vi "Laser Ablation and Capture.vi"() -> ()   [LabVIEW 2016] (continued)
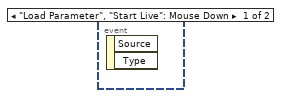
[diagram p2: hidden frame]
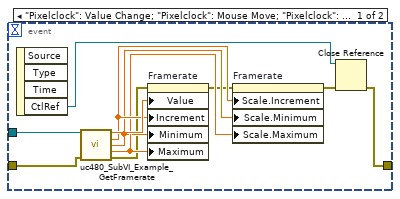
[diagram p3: hidden frame]
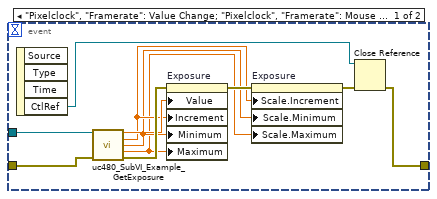
[diagram p4: hidden frame]
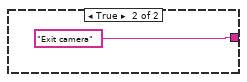
[diagram p5: hidden frame]
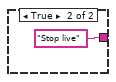
[diagram p6: hidden frame]
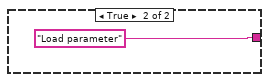
[diagram p7: hidden frame]
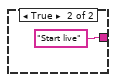
[diagram p8: hidden frame]
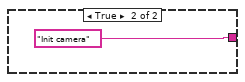
[diagram p9: hidden frame]
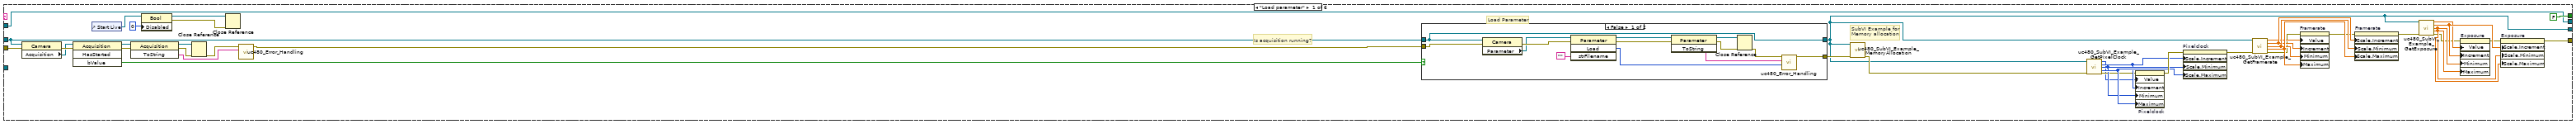
[diagram p10: hidden frame]
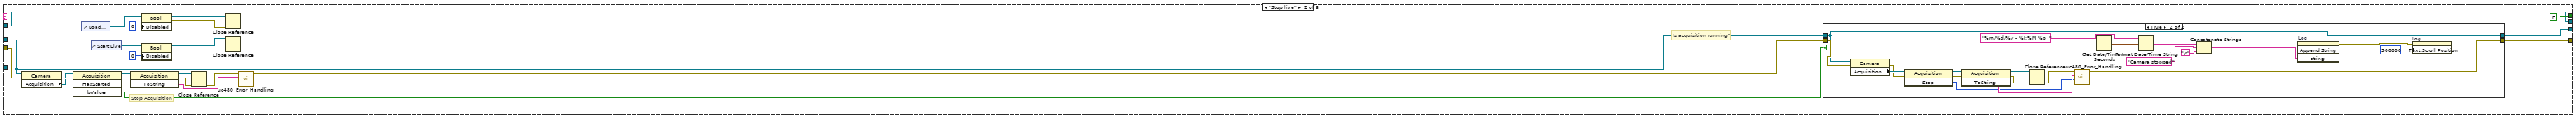
[diagram p12: hidden frame]
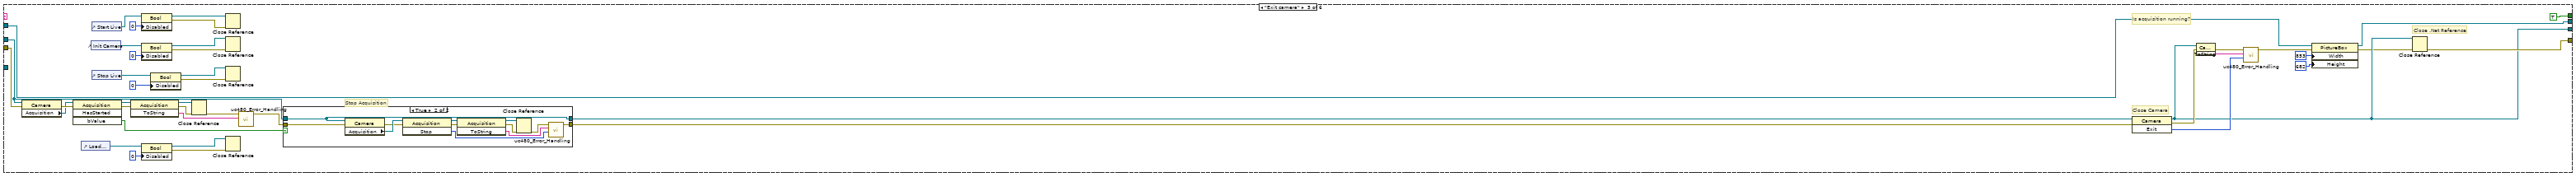
[diagram p14: hidden frame]
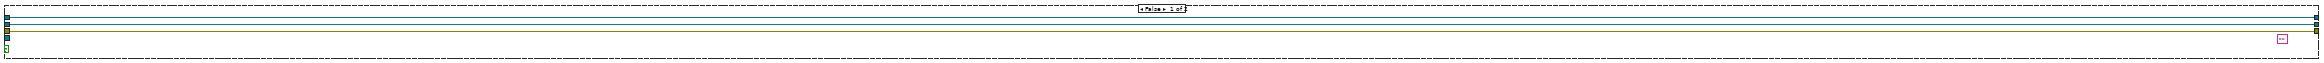
[diagram p16: hidden frame]
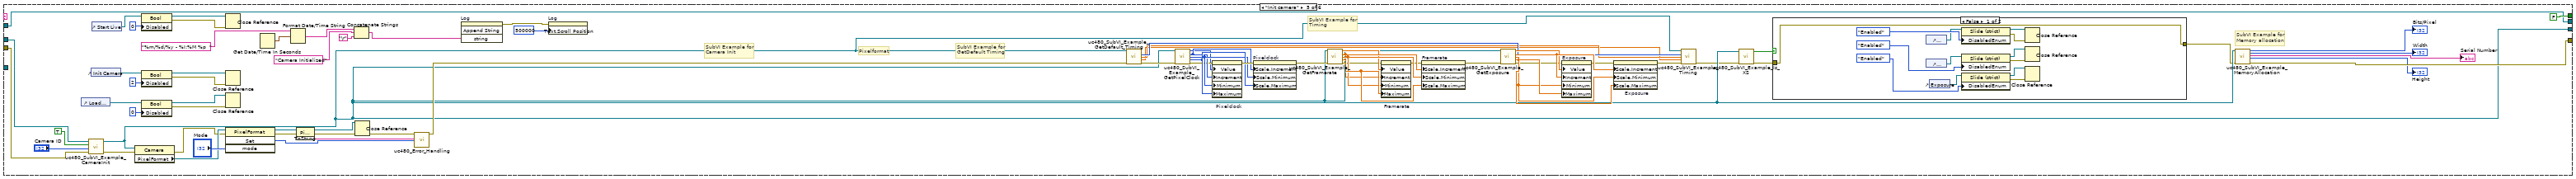
[diagram p18: hidden frame]
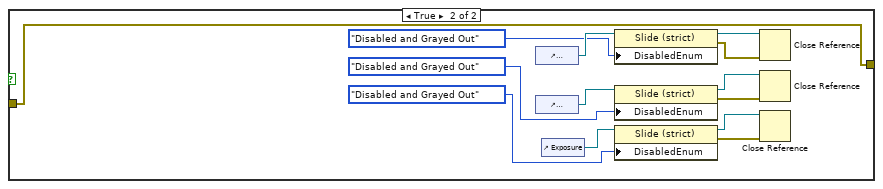
[diagram p19: hidden frame]
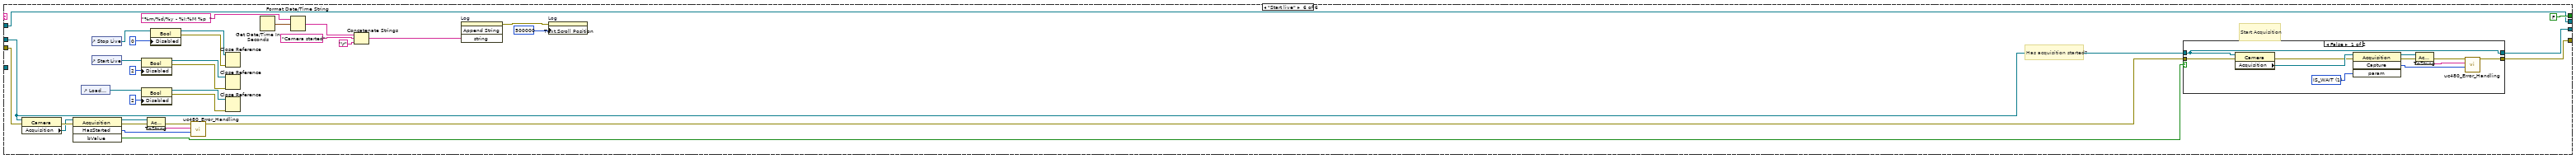
[diagram p20: hidden frame]
            n599 = case shown="False" w1486 {
              tunnel: w1485 -> [w1497 _]
              frame False {
                n600 = call "IMAQ Create"("Image Name"="untitled") -> ("New Image"=w1499:T2)  [unwired: 4 in, 1 out]
                n601 = call "IMAQ ReadFile"("File Path"=w1497, "Image"=w1499) -> ("Image Out"=w1498:T2)  [unwired: 5 in, 4 out]
                n602 = call "IMAQ MaskToROI"("Image"=w1498) -> ("ROI Descriptor"=w1490:T11)  [unwired: 6 in, 2 out]
                n603 = Unbundle By Name(w1490) -> ("Contours"=w1495:T12)  [unwired: 1 out]
                n604 = Index Array(array=w1495) -> (element=w1496:T13)  [unwired: 1 in]
                n605 = Bundle By Name(cluster=w1496, "Type"=u32 6) -> (w1494:T13)
                n606 = Replace Array Subset(array=w1495, new element=w1494) -> (w1493:T12)  [unwired: 1 in]
                n607 = Bundle By Name(cluster=w1490, "Contours"=w1493) -> (w1491:T11)
                n608 = property on="Source" class="ImageControl"("ROI"=w1491) -> ()  [unwired: 2 in, 2 out]
              }
              frame True {
              }
            }
          }
        }
      }
      event "Axes Manual Control": Value Change {
        n609 = event-data() -> ()  [unwired: 1 in, 6 out]
        n610 = case shown="True" "Axes Manual Control" {
          tunnel: w1503 -> [_ w1515]
          tunnel: w1502 -> [_ w1514]
          tunnel: w1501 -> [_ w1513]
          frame False {
          }
          frame True {
            n611 = flat-sequence {
              tunnel: w1515 -> [w1525]
              tunnel: w1514 -> [w1524]
              tunnel: w1513 -> [w1523]
              tunnel: [w1525] -> w1512
              tunnel: [w1524] -> w1511
              tunnel: [w1523] -> w1510
              tunnel: [w1522] -> w1509
              tunnel: [w1521] -> w1508
              tunnel: [w1520] -> w1507
              tunnel: [w1519] -> w1506
              tunnel: w1512 -> [w1568]
              tunnel: w1511 -> [w1567]
              tunnel: w1510 -> [w1566]
              tunnel: w1509 -> [w1561]
              tunnel: w1508 -> [w1560]
              tunnel: w1507 -> [w1551]
              tunnel: w1506 -> [w1550]
              frame #0 {
                n612 = call <userlib>:"Open TCP-IP.vi"("IP address"=w1525) -> ("error out"=w1517:errorcluster, "Connection ID"=w1526:T9)  [unwired: 8 in, 1 out]
                n613 = call <vilib>:"Simple Error Handler.vi"("error in (no error)"=w1517) -> ("error?"=w1516:bool, "error out"=w1518:errorcluster)  [unwired: 4 in, 3 out]
                n614 = case shown="True" w1516 {
                  tunnel: w1526 -> [w1541 _]
                  tunnel: w1518 -> [w1540 _]
                  tunnel: w1524 -> [w1537 _]
                  tunnel: w1523 -> [w1536 _]
                  tunnel: [w1535 w1545] -> w1522
                  tunnel: [w1534 w1545] -> w1521
                  tunnel: [w1530 w1544] -> w1520
                  tunnel: [w1529 w1544] -> w1519
                  frame False {
                    n615 = call "Get Stages Status.vi"("error in (no error)"=w1540, "Group Name (250 c max)"=w1537, "connection ID in"=w1541) -> ("error out"=w1539:errorcluster, "XPS error out"=w1538:errorcluster, "Group Status String"=w1534:string, "connection ID out"=w1533:T9, "Status"=w1529:i32)  [unwired: 4 in]
                    n616 = call "Get Stages Status.vi"("error in (no error)"=w1539, "XPS error in (no error)"=w1538, "Group Name (250 c max)"=w1536, "connection ID in"=w1533) -> ("error out"=w1543:errorcluster, "XPS error out"=w1532:errorcluster, "Group Status String"=w1535:string, "connection ID out"=w1542:T9, "Status"=w1530:i32)  [unwired: 3 in]
                    n617 = call <vilib>:"Simple Error Handler.vi"("error source (\" \")"="Axis manual control check" ("error source (\" \")"), "error in (no error)"=w1532) -> ()  [unwired: 3 in, 5 out]
                    n618 = call <userlib>:"Close TCP-IP.vi"("error in (no error)"=w1543, "connection ID in"=w1542) -> ("Error out"=w1531:errorcluster)  [unwired: 9 in]
                    n619 = call <vilib>:"Simple Error Handler.vi"("error source (\" \")"="TCP close Axis manual control check" ("error source (\" \")"), "error in (no error)"=w1531) -> ()  [unwired: 3 in, 5 out]
                  }
                  frame True {
                    w1544 = 0
                    w1545 = ""
                  }
                }
              }
              frame #1 {
                w1554 = 47 ("y")
                w1555 = "Ready"
                n620 = String Subset(string=w1560, offset (0)=0, length (rest)=5 ("length (rest)")) -> (substring=w1557:string)
                n621 = String Subset(string=w1561, offset (0)=0, length (rest)=5 ("length (rest)")) -> (substring=w1556:string)
                n622 = Equal?(x=w1557, y=w1555) -> (x = y?=w1558:bool)
                n623 = Equal?(x=w1555, y=w1556) -> (x = y?=w1559:bool)
                n624 = Equal?(x=w1554, y=w1550) -> (x = y?=w1552:bool)
                n625 = Equal?(x=w1551, y=w1554) -> (x = y?=w1553:bool)
                n626 = And(x=w1553, y=w1552) -> (x .and. y?=w1547:bool)
                n627 = And(x=w1558, y=w1559) -> (x .and. y?=w1548:bool)
                n628 = Not(x=w1547) -> (.not. x?=w1546:bool)
                n629 = And(x=w1548, y=w1546) -> (x .and. y?=w1549:bool)
                n630 = case shown="True" w1549 {
                  tunnel: w1568 -> [_ w1576]
                  tunnel: w1567 -> [_ w1575]
                  tunnel: w1566 -> [_ w1574]
                  tunnel: w1546 -> [w1569 _]
                  frame False {
                    n631 = case shown="False" w1569 {
                      frame False {
                        n632 = One Button Dialog(message="One or more axis already in jogging position") -> ()  [unwired: 1 in, 1 out]
                      }
                      frame True {
                        n633 = One Button Dialog(message="Axes are not ready") -> ()  [unwired: 1 in, 1 out]
                      }
                    }
                  }
                  frame True {
                    n634 = local read "Axis 2 inverted?"() -> (w1573:bool)
                    n635 = local read "Axis 1 inverted?"() -> (w1572:bool)
                    n636 = call "XPS Controller.vi"("Axis 2"=w1574, "Axis 1"=w1575, "Controller Address"=w1576, "Axis 2 \ninverted?"=w1573, "Axis 1 \ninverted?"=w1572) -> ()  [unwired: 6 in]
                  }
                }
              }
            }
          }
        }
      }
      event "Home Axes": Value Change {
        n637 = event-data() -> ()  [unwired: 1 in, 6 out]
        n638 = flat-sequence {
          tunnel: w1583 -> [w1589]
          tunnel: w1584 -> [w1590]
          tunnel: w1585 -> [w1591]
          tunnel: "Home Axes" -> [w1592]
          tunnel: [w1592] -> w1581
          tunnel: [w1591] -> w1580
          tunnel: [w1590] -> w1579
          tunnel: [w1589] -> w1578
          tunnel: [w1588] -> w1577
          tunnel: [w1596] -> w1582
          tunnel: w1581 -> [w1594]
          tunnel: w1580 -> [w1599]
          tunnel: w1579 -> [w1597]
          tunnel: w1578 -> [w1598]
          tunnel: w1577 -> [w1595]
          tunnel: [w1678] -> w1586
          tunnel: w1582 -> [w1677]
          frame #0 {
            n639 = call "Display Message to User"() -> ("OK"=w1588:bool)  [unwired: 10 in, 1 out]
          }
          frame #1 {
            n640 = And(x=w1594, y=w1595) -> (x .and. y?=w1593:bool)
            n641 = case shown="True" w1593 {
              tunnel: w1599 -> [_ w1615]
              tunnel: w1597 -> [_ w1616]
              tunnel: w1598 -> [_ w1613]
              tunnel: w1597 -> [_ w1614]
              tunnel: [FALSE w1606] -> w1596
              frame False {
              }
              frame True {
                w1612 = 47 ("y")
                w1628 = "Ready"
                n642 = call <userlib>:"Open TCP-IP.vi"("IP address"=w1615) -> ("error out"=w1601:errorcluster, "Connection ID"=w1619:T9)  [unwired: 8 in, 1 out]
                n643 = call <vilib>:"Simple Error Handler.vi"("error in (no error)"=w1601) -> ("error?"=w1603:bool, "error out"=w1602:errorcluster)  [unwired: 4 in, 3 out]
                n644 = case shown="False" w1603 {
                  tunnel: w1602 -> [w1642 _]
                  tunnel: w1619 -> [w1641 _]
                  tunnel: [w1638 w1647] -> w1618
                  tunnel: [w1637 w1647] -> w1617
                  tunnel: w1616 -> [w1636 _]
                  tunnel: w1613 -> [w1635 _]
                  tunnel: [w1632 w1646] -> w1611
                  tunnel: [w1631 w1646] -> w1610
                  frame False {
                    n645 = call "Get Stages Status.vi"("error in (no error)"=w1642, "Group Name (250 c max)"=w1636, "connection ID in"=w1641) -> ("error out"=w1643:errorcluster, "XPS error out"=w1644:errorcluster, "Group Status String"=w1638:string, "connection ID out"=w1645:T9, "Status"=w1631:i32)  [unwired: 4 in]
                    n646 = call "Get Stages Status.vi"("error in (no error)"=w1643, "XPS error in (no error)"=w1644, "Group Name (250 c max)"=w1635, "connection ID in"=w1645) -> ("error out"=w1639:errorcluster, "XPS error out"=w1634:errorcluster, "Group Status String"=w1637:string, "connection ID out"=w1640:T9, "Status"=w1632:i32)  [unwired: 3 in]
                    n647 = call <vilib>:"Simple Error Handler.vi"("error source (\" \")"="home axis check" ("error source (\" \")"), "error in (no error)"=w1634) -> ()  [unwired: 3 in, 5 out]
                    n648 = call <userlib>:"Close TCP-IP.vi"("error in (no error)"=w1639, "connection ID in"=w1640) -> ("Error out"=w1633:errorcluster)  [unwired: 9 in]
                    n649 = call <vilib>:"Simple Error Handler.vi"("error source (\" \")"="TCP close home axis check" ("error source (\" \")"), "error in (no error)"=w1633) -> ()  [unwired: 3 in, 5 out]
                  }
                  frame True {
                    w1646 = 0
                    w1647 = ""
                  }
                }
                n650 = Equal?(x=w1612, y=w1610) -> (x = y?=w1609:bool)
                n651 = Equal?(x=w1611, y=w1612) -> (x = y?=w1608:bool)
                n652 = String Subset(string=w1618, offset (0)=0, length (rest)=5 ("length (rest)")) -> (substring=w1626:string)
                n653 = String Subset(string=w1617, offset (0)=0, length (rest)=5 ("length (rest)")) -> (substring=w1627:string)
                n654 = Equal?(x=w1626, y=w1628) -> (x = y?=w1625:bool)
                n655 = Equal?(x=w1628, y=w1627) -> (x = y?=w1624:bool)
                n656 = And(x=w1608, y=w1609) -> (x .and. y?=w1604:bool)
                n657 = Not(x=w1604) -> (.not. x?=w1605:bool)
                n658 = And(x=w1625, y=w1624) -> (x .and. y?=w1607:bool)
                n659 = And(x=w1607, y=w1605) -> (x .and. y?=w1606:bool)
                n660 = case shown="True" w1606 {
                  tunnel: w1615 -> [_ w1657]
                  tunnel: w1614 -> [_ w1656]
                  tunnel: w1613 -> [_ w1655]
                  tunnel: w1604 -> [w1648 _]
                  frame False {
                    n661 = case shown="True" w1648 {
                      frame False {
                        n662 = One Button Dialog(message="Axes are not ready") -> ()  [unwired: 1 in, 1 out]
                      }
                      frame True {
                        n663 = One Button Dialog(message="One or more axis are in jogging mode") -> ()  [unwired: 1 in, 1 out]
                      }
                    }
                  }
                  frame True {
                    n664 = call <userlib>:"Open TCP-IP.vi"("IP address"=w1657) -> ("error out"=w1673:errorcluster, "Connection ID"=w1674:T9)  [unwired: 8 in, 1 out]
                    n665 = call <userlib>:"Group Kill.vi"("error in (no error)"=w1673, "Group Name (250 c max)"=w1656, "connection ID in"=w1674) -> ("error out"=w1671:errorcluster, "XPS error out"=w1672:errorcluster, "connection ID out"=w1668:T9)  [unwired: 6 in]
                    n666 = call <userlib>:"Group Initialize.vi"("error in (no error)"=w1671, "XPS error in (no error)"=w1672, "Group Name (250 c max)"=w1656, "connection ID in"=w1668) -> ("error out"=w1669:errorcluster, "XPS error out"=w1670:errorcluster, "connection ID out"=w1667:T9)  [unwired: 5 in]
                    n667 = call <userlib>:"Group Home Search.vi"("error in (no error)"=w1669, "XPS error in (no error)"=w1670, "Group Name (250 c max)"=w1656, "connection ID in"=w1667) -> ("error out"=w1658:errorcluster, "XPS error out"=w1659:errorcluster, "connection ID out"=w1666:T9)  [unwired: 5 in]
                    n668 = call <userlib>:"Group Kill.vi"("error in (no error)"=w1658, "XPS error in (no error)"=w1659, "Group Name (250 c max)"=w1655, "connection ID in"=w1666) -> ("error out"=w1660:errorcluster, "XPS error out"=w1661:errorcluster, "connection ID out"=w1665:T9)  [unwired: 5 in]
                    n669 = call <userlib>:"Group Initialize.vi"("error in (no error)"=w1660, "XPS error in (no error)"=w1661, "Group Name (250 c max)"=w1655, "connection ID in"=w1665) -> ("error out"=w1662:errorcluster, "XPS error out"=w1663:errorcluster, "connection ID out"=w1664:T9)  [unwired: 5 in]
                    n670 = call <userlib>:"Group Home Search.vi"("error in (no error)"=w1662, "XPS error in (no error)"=w1663, "Group Name (250 c max)"=w1655, "connection ID in"=w1664) -> ("error out"=w1675:errorcluster, "XPS error out"=w1654:errorcluster, "connection ID out"=w1676:T9)  [unwired: 5 in]
                    n671 = call <vilib>:"Simple Error Handler.vi"("error source (\" \")"="home axis " ("error source (\" \")"), "error in (no error)"=w1654) -> ()  [unwired: 3 in, 5 out]
                    n672 = call <userlib>:"Close TCP-IP.vi"("error in (no error)"=w1675, "connection ID in"=w1676) -> ("Error out"=w1653:errorcluster)  [unwired: 9 in]
                    n673 = call <vilib>:"Simple Error Handler.vi"("error source (\" \")"="TCP close home axis " ("error source (\" \")"), "error in (no error)"=w1653) -> ()  [unwired: 3 in, 5 out]
                  }
                }
              }
            }
          }
          frame #2 {
            n674 = case shown="True" w1677 {
              tunnel: ["" ("StringOut") "Axes have been moved to home position" ("StringOut")] -> w1678
              frame False {
              }
              frame True {
              }
            }
          }
        }
      }
      event "Transparency": Value Change {
        n675 = event-data() -> ()  [unwired: 1 in, 6 out]
        n676 = control-ref of="This VI"() -> (w1682:refnum<vi>)
        n677 = property class="VI"(reference=w1682, "FP:Transparency"="Transparency") -> ()  [unwired: 1 in, 2 out]
      }
      event "Capture": Value Change {
        w1683 = 47 ("y")
        w1709 = "Ready"
        n678 = event-data() -> ()  [unwired: 1 in, 6 out]
        n679 = call <userlib>:"Open TCP-IP.vi"("IP address"=w1697) -> ("error out"=w1686:errorcluster, "Connection ID"=w1700:T9)  [unwired: 8 in, 1 out]
        n680 = call <vilib>:"Simple Error Handler.vi"("error in (no error)"=w1686) -> ("error?"=w1684:bool, "error out"=w1685:errorcluster)  [unwired: 4 in, 3 out]
        n681 = case shown="False" w1684 {
          tunnel: w1685 -> [w1723 _]
          tunnel: w1700 -> [w1722 _]
          tunnel: [w1719 w1727] -> w1699
          tunnel: [w1718 w1727] -> w1698
          tunnel: w1696 -> [w1717 _]
          tunnel: w1695 -> [w1716 _]
          tunnel: [w1714 w1728] -> w1694
          tunnel: [w1713 w1728] -> w1693
          frame False {
            n682 = call "Get Stages Status.vi"("error in (no error)"=w1723, "Group Name (250 c max)"=w1717, "connection ID in"=w1722) -> ("error out"=w1724:errorcluster, "XPS error out"=w1725:errorcluster, "Group Status String"=w1719:string, "connection ID out"=w1726:T9, "Status"=w1713:i32)  [unwired: 4 in]
            n683 = call "Get Stages Status.vi"("error in (no error)"=w1724, "XPS error in (no error)"=w1725, "Group Name (250 c max)"=w1716, "connection ID in"=w1726) -> ("error out"=w1720:errorcluster, "XPS error out"=w1715:errorcluster, "Group Status String"=w1718:string, "connection ID out"=w1721:T9, "Status"=w1714:i32)  [unwired: 3 in]
            n684 = call <vilib>:"Simple Error Handler.vi"("error source (\" \")"="Capture check" ("error source (\" \")"), "error in (no error)"=w1715) -> ()  [unwired: 3 in, 5 out]
            n685 = call <userlib>:"Close TCP-IP.vi"("error in (no error)"=w1720, "connection ID in"=w1721) -> ("Error out"=w1711:errorcluster)  [unwired: 9 in]
            n686 = call <vilib>:"Simple Error Handler.vi"("error in (no error)"=w1711) -> ()  [unwired: 4 in, 5 out]
          }
          frame True {
            w1728 = 0
            w1727 = ""
          }
        }
        n687 = Equal?(x=w1694, y=w1683) -> (x = y?=w1692:bool)
        n688 = Equal?(x=w1683, y=w1693) -> (x = y?=w1691:bool)
        n689 = String Subset(string=w1699, offset (0)=0, length (rest)=5 ("length (rest)")) -> (substring=w1707:string)
        n690 = String Subset(string=w1698, offset (0)=0, length (rest)=5 ("length (rest)")) -> (substring=w1708:string)
        n691 = Equal?(x=w1707, y=w1709) -> (x = y?=w1706:bool)
        n692 = Equal?(x=w1709, y=w1708) -> (x = y?=w1705:bool)
        n693 = And(x=w1692, y=w1691) -> (x .and. y?=w1688:bool)
        n694 = Not(x=w1688) -> (.not. x?=w1687:bool)
        n695 = And(x=w1706, y=w1705) -> (x .and. y?=w1690:bool)
        n696 = And(x=w1690, y=w1687) -> (x .and. y?=w1689:bool)
        n697 = case shown="True" w1689 {
          tunnel: ["" w1754] -> w1710
          tunnel: w1697 -> [_ w1753]
          tunnel: w1695 -> [_ w1752]
          tunnel: w1696 -> [_ w1751]
          tunnel: w1688 -> [w1729 _]
          frame False {
            n698 = case shown="True" w1729 {
              frame False {
                n699 = One Button Dialog(message="Axes are not ready") -> ()  [unwired: 1 in, 1 out]
              }
              frame True {
                n700 = One Button Dialog(message="One or more axis are in jogging mode") -> ()  [unwired: 1 in, 1 out]
              }
            }
          }
          frame True {
            n701 = flat-sequence {
              tunnel: [w1784] -> w1765
              tunnel: [w1770] -> w1764
              tunnel: [w1769] -> w1763
              tunnel: [w1783] -> w1762
              tunnel: [w1782] -> w1761
              tunnel: [w1781] -> w1760
              tunnel: [w1768] -> w1759
              tunnel: w1751 -> [w1779]
              tunnel: w1752 -> [w1780]
              tunnel: w1753 -> [w1768]
              tunnel: [w1767] -> w1740
              tunnel: [w1766] -> w1736
              tunnel: w1765 -> [w1804]
              tunnel: w1764 -> [w1792]
              tunnel: w1763 -> [w1791]
              tunnel: w1762 -> [w1802]
              tunnel: w1761 -> [w1801]
              tunnel: [w1796] -> w1758
              tunnel: w1760 -> [w1796]
              tunnel: [w1795] -> w1757
              tunnel: w1759 -> [w1795]
              tunnel: [w1792] -> w1750
              tunnel: [w1791] -> w1748
              tunnel: [w1790] -> w1741
              tunnel: w1740 -> [w1790]
              tunnel: [w1789] -> w1737
              tunnel: w1736 -> [w1789]
              tunnel: [w1810] -> w1756
              tunnel: w1758 -> [w1810]
              tunnel: [w1809] -> w1755
              tunnel: w1757 -> [w1809]
              tunnel: w1750 -> [w1808]
              tunnel: [w1808] -> w1749
              tunnel: w1748 -> [w1807]
              tunnel: [w1807] -> w1747
              tunnel: [w1806] -> w1742
              tunnel: w1741 -> [w1806]
              tunnel: [w1805] -> w1738
              tunnel: w1737 -> [w1805]
              tunnel: w1756 -> [w1824]
              tunnel: w1755 -> [w1814]
              tunnel: [w1823] -> w1746
              tunnel: w1749 -> [w1813]
              tunnel: w1747 -> [w1812]
              tunnel: [w1817] -> w1744
              tunnel: [w1816] -> w1743
              tunnel: w1742 -> [w1816]
              tunnel: [w1815] -> w1739
              tunnel: w1738 -> [w1815]
              tunnel: [w1814] -> w1735
              tunnel: [w1813] -> w1734
              tunnel: [w1812] -> w1733
              tunnel: w1746 -> [w1846]
              tunnel: [w1846] -> w1745
              tunnel: w1744 -> [w1842]
              tunnel: w1743 -> [w1836]
              tunnel: w1739 -> [w1835]
              tunnel: w1735 -> [w1840]
              tunnel: w1734 -> [w1834]
              tunnel: w1733 -> [w1833]
              tunnel: [w1851] -> w1754
              tunnel: w1745 -> [w1848]
              frame #0 {
                w1788 = ".Pos"
                n702 = call <userlib>:"Open TCP-IP.vi"("IP address"=w1768) -> ("error out"=w1773:errorcluster, "Connection ID"=w1775:T9)  [unwired: 5 in, 4 out]
                n703 = Concatenate Strings(w1780, w1788) -> (w1769:string)
                n704 = Concatenate Strings(w1779, w1788) -> (w1770:string)
                n705 = call <userlib>:"Single Axis Group Position Current Get.vi"("error in (no error)"=w1773, "SingleAxis Group  Name (250 c max)"=w1770, "connection ID in"=w1775) -> ("error out"=w1776:errorcluster, "XPS error out"=w1777:errorcluster, "Current Position (units)"=w1766:dbl, "connection ID out"=w1778:T9)  [unwired: 5 in]
                "Pre-Capture Axis 1" <- w1766
                n706 = call <userlib>:"Single Axis Group Position Current Get.vi"("error in (no error)"=w1776, "XPS error in (no error)"=w1777, "SingleAxis Group  Name (250 c max)"=w1769, "connection ID in"=w1778) -> ("error out"=w1772:errorcluster, "XPS error out"=w1771:errorcluster, "Current Position (units)"=w1767:dbl, "connection ID out"=w1774:T9)  [unwired: 4 in]
                "Pre-Capture Axis 2" <- w1767
                n707 = local read "Axis Initial Parameters"() -> (w1781:T1)
                n708 = call <userlib>:"Positioner SGamma Parameters Set.vi"("SGamma Parameters"=w1781, "error in (no error)"=w1772, "XPS error in (no error)"=w1771, "Positioner Name (250 c max)"=w1770, "connection ID in"=w1774) -> ("error out"=w1785:errorcluster, "XPS error out"=w1786:errorcluster, "connection ID out"=w1787:T9)  [unwired: 4 in]
                n709 = call <userlib>:"Positioner SGamma Parameters Set.vi"("SGamma Parameters"=w1781, "error in (no error)"=w1785, "XPS error in (no error)"=w1786, "Positioner Name (250 c max)"=w1769, "connection ID in"=w1787) -> ("error out"=w1783:errorcluster, "XPS error out"=w1782:errorcluster, "connection ID out"=w1784:T9)  [unwired: 4 in]
              }
              frame #1 {
                n710 = local read "Axis 1 Offset"() -> (w1794:dbl)
                n711 = local read "Axis 2 Offset"() -> (w1793:dbl)
                n712 = call <userlib>:"Single Axis Group Move Relative.vi"("Target Displacement (units)"=w1794, "error in (no error)"=w1802, "XPS error in (no error)"=w1801, "SingleAxis Group  Name (250 c max)"=w1792, "connection ID in"=w1804) -> ("error out"=w1799:errorcluster, "XPS error out"=w1800:errorcluster, "connection ID out"=w1803:T9)  [unwired: 4 in]
                n713 = call <userlib>:"Single Axis Group Move Relative.vi"("Target Displacement (units)"=w1793, "error in (no error)"=w1799, "XPS error in (no error)"=w1800, "SingleAxis Group  Name (250 c max)"=w1791, "connection ID in"=w1803) -> ("error out"=w1797:errorcluster, "connection ID out"=w1798:T9)  [unwired: 4 in, 1 out]
                n714 = call <userlib>:"Close TCP-IP.vi"("error in (no error)"=w1797, "connection ID in"=w1798) -> ()  [unwired: 9 in, 1 out]
              }
              frame #2 {
                n715 = Wait (ms)(milliseconds to wait=u32 1000) -> ()  [unwired: 1 out]
              }
              frame #3 {
                n716 = local read "Speed (µm/s)"() -> (w1828:i32)
                n717 = local read "Processi time (sec)"() -> (w1822:i32)
                n718 = local read "Laser on/off array"() -> (w1831:bool[][])
                n719 = local read "Commands array"() -> (w1832:string[][])
                n720 = local read "ROI Area \n(mm2)"() -> (w1820:dbl)
                n721 = local read "Laser Com Delay"() -> (w1819:i32)
                n722 = local read "VISA Laser port"() -> (w1818:string)
                n723 = Divide(x=w1828, y=1000) -> (x/y=w1825:dbl)
                n724 = call "Capture.vi"("Commands array"=w1832, "XPS_Address"=w1814, "VISA resource name"=w1818, "laser array index"=0, "Process time"=w1822, "Axis Speed"=w1825, "Laser on/off array"=w1831, "stop"=FALSE ("STOP CAPTURE"), "delay before read (ms)"=w1819, "Axis Initial Parameters"=w1824, "ROI Area \n(mm2)"=w1820, "Axis 2"=w1812, "Axis 1"=w1813, "OPO on?"=TRUE, "Acceleration (units/seconds²)"="Acceleration \n(mm/s²)") -> ("Elapsed time"=w1823:dbl, "XPS error out"=w1817:errorcluster)  [unwired: 2 in, 1 out]
              }
              frame #4 {
                n725 = call <userlib>:"Open TCP-IP.vi"("IP address"=w1840) -> ("error out"=w1839:errorcluster, "Connection ID"=w1841:T9)  [unwired: 5 in, 4 out]
                n726 = call <userlib>:"Single Axis Group Move Absolute.vi"("Target Position (units)"=w1835, "error in (no error)"=w1839, "XPS error in (no error)"=w1842, "SingleAxis Group  Name (250 c max)"=w1834, "connection ID in"=w1841) -> ("error out"=w1844:errorcluster, "XPS error out"=w1843:errorcluster, "connection ID out"=w1845:T9)  [unwired: 4 in]
                n727 = call <userlib>:"Single Axis Group Move Absolute.vi"("Target Position (units)"=w1836, "error in (no error)"=w1844, "XPS error in (no error)"=w1843, "SingleAxis Group  Name (250 c max)"=w1833, "connection ID in"=w1845) -> ("error out"=w1837:errorcluster, "connection ID out"=w1838:T9)  [unwired: 4 in, 1 out]
                n728 = call <userlib>:"Close TCP-IP.vi"("error in (no error)"=w1837, "connection ID in"=w1838) -> ()  [unwired: 9 in, 1 out]
              }
              frame #5 {
                n729 = Number To Decimal String(number=w1848) -> (decimal integer string=w1847:string)  [unwired: 1 in]
                n730 = Concatenate Strings("Capture completed in " ("StringOut"), w1847, " seconds" ("string")) -> (w1851:string)
              }
            }
          }
        }
      }
      event "Microscope/Capture \nstatus button": Value Change {
        w1871 = 47 ("y")
        w1884 = "Ready"
        n731 = event-data() -> ()  [unwired: 1 in, 6 out]
        n732 = call <userlib>:"Open TCP-IP.vi"("IP address"=w1854) -> ("error out"=w1887:errorcluster, "Connection ID"=w1888:T9)  [unwired: 8 in, 1 out]
        n733 = call <vilib>:"Simple Error Handler.vi"("error in (no error)"=w1887) -> ("error?"=w1885:bool, "error out"=w1886:errorcluster)  [unwired: 4 in, 3 out]
        n734 = case shown="False" w1885 {
          tunnel: w1888 -> [w1966 _]
          tunnel: [w1963 w1970] -> w1870
          tunnel: [w1962 w1970] -> w1869
          tunnel: w1864 -> [w1961 _]
          tunnel: w1865 -> [w1960 _]
          tunnel: [w1958 w1971] -> w1868
          tunnel: [w1957 w1971] -> w1867
          tunnel: w1886 -> [w1954 _]
          frame False {
            n735 = call "Get Stages Status.vi"("error in (no error)"=w1954, "Group Name (250 c max)"=w1961, "connection ID in"=w1966) -> ("error out"=w1967:errorcluster, "XPS error out"=w1968:errorcluster, "Group Status String"=w1963:string, "connection ID out"=w1969:T9, "Status"=w1957:i32)  [unwired: 4 in]
            n736 = call "Get Stages Status.vi"("error in (no error)"=w1967, "XPS error in (no error)"=w1968, "Group Name (250 c max)"=w1960, "connection ID in"=w1969) -> ("error out"=w1964:errorcluster, "XPS error out"=w1959:errorcluster, "Group Status String"=w1962:string, "connection ID out"=w1965:T9, "Status"=w1958:i32)  [unwired: 3 in]
            n737 = call <vilib>:"Simple Error Handler.vi"("error source (\" \")"="Axes check" ("error source (\" \")"), "error in (no error)"=w1959) -> ()  [unwired: 3 in, 5 out]
            n738 = call <userlib>:"Close TCP-IP.vi"("error in (no error)"=w1964, "connection ID in"=w1965) -> ("Error out"=w1955:errorcluster)  [unwired: 9 in]
            n739 = call <vilib>:"Simple Error Handler.vi"("error in (no error)"=w1955) -> ()  [unwired: 4 in, 5 out]
          }
          frame True {
            w1971 = 0
            w1970 = ""
          }
        }
        n740 = Equal?(x=w1868, y=w1871) -> (x = y?=w1875:bool)
        n741 = Equal?(x=w1871, y=w1867) -> (x = y?=w1874:bool)
        n742 = String Subset(string=w1870, offset (0)=0, length (rest)=5 ("length (rest)")) -> (substring=w1882:string)
        n743 = String Subset(string=w1869, offset (0)=0, length (rest)=5 ("length (rest)")) -> (substring=w1883:string)
        n744 = case shown="False" "Microscope/Capture \nstatus button" {
          tunnel: ["capture " "microscope "] -> w1858
          frame False {
          }
          frame True {
          }
        }
        n745 = Equal?(x=w1882, y=w1884) -> (x = y?=w1881:bool)
        n746 = Equal?(x=w1884, y=w1883) -> (x = y?=w1880:bool)
        n747 = And(x=w1875, y=w1874) -> (x .and. y?=w1866:bool)
        n748 = Not(x=w1866) -> (.not. x?=w1872:bool)
        n749 = And(x=w1881, y=w1880) -> (x .and. y?=w1873:bool)
        n750 = And(x=w1873, y=w1872) -> (x .and. y?=w1856:bool)
        n751 = Concatenate Strings("Do you want to move the axis to the " ("message"), w1858, "position?" ("string")) -> (w1857:string)
        n752 = Two Button Dialog(message=w1857, 1:"No" ("F button name (\"Cancel\")"), 2:"Yes" ("T button name (\"OK\")")) -> (T button?=w1853:bool)
        n753 = case shown="False" w1853 {
          tunnel: "Microscope/Capture \nstatus button" -> [w1889 _]
          frame False {
            n754 = Not(x=w1889) -> (.not. x?=w1890:bool)
            n755 = local write "Microscope/Capture \nstatus button"(w1890) -> ()
          }
          frame True {
          }
        }
        n756 = And(x=w1856, y=w1853) -> (x .and. y?=w1855:bool)
        n757 = case shown="True" w1855 {
          tunnel: "Microscope/Capture \nstatus button" -> [w1894 w1899]
          tunnel: w1866 -> [w1895 _]
          tunnel: w1865 -> [_ w1907]
          tunnel: w1864 -> [_ w1906]
          tunnel: [_ w1905] -> w1863
          tunnel: w1854 -> [_ w1898]
          frame False {
            n758 = Not(x=w1894) -> (.not. x?=w1893:bool)
            n759 = case shown="True" w1895 {
              frame False {
                n760 = One Button Dialog(message="Axes are not ready") -> ()  [unwired: 1 in, 1 out]
              }
              frame True {
                n761 = One Button Dialog(message="One or more axis are in jogging mode") -> ()  [unwired: 1 in, 1 out]
              }
            }
            n762 = local write "Microscope/Capture \nstatus button"(w1893) -> ()
          }
          frame True {
            n763 = flat-sequence {
              tunnel: [w1918] -> w1904
              tunnel: [w1917] -> w1903
              tunnel: [w1916] -> w1902
              tunnel: [w1915] -> w1901
              tunnel: [w1914] -> w1900
              tunnel: w1907 -> [w1913]
              tunnel: w1906 -> [w1912]
              tunnel: w1898 -> [w1911]
              tunnel: w1904 -> [w1939]
              tunnel: w1903 -> [w1930]
              tunnel: w1902 -> [w1931]
              tunnel: w1901 -> [w1937]
              tunnel: w1900 -> [w1936]
              tunnel: w1899 -> [w1925]
              tunnel: [w1951] -> w1905
              tunnel: w1899 -> [w1947]
              frame #0 {
                w1923 = ".Pos"
                n764 = local read "Axis Initial Parameters"() -> (w1910:T1)
                n765 = Bundle By Name(cluster=w1910, "Velocity (units/seconds)"=10.0) -> (w1908:T1)
                n766 = call <userlib>:"Open TCP-IP.vi"("IP address"=w1911) -> ("error out"=w1919:errorcluster, "Connection ID"=w1924:T9)  [unwired: 5 in, 4 out]
                n767 = Concatenate Strings(w1912, w1923) -> (w1917:string)
                n768 = call <userlib>:"Positioner SGamma Parameters Set.vi"("SGamma Parameters"=w1910, "error in (no error)"=w1919, "Positioner Name (250 c max)"=w1917, "connection ID in"=w1924) -> ("error out"=w1920:errorcluster, "XPS error out"=w1921:errorcluster, "connection ID out"=w1922:T9)  [unwired: 5 in]
                n769 = Concatenate Strings(w1913, w1923) -> (w1916:string)
                n770 = call <userlib>:"Positioner SGamma Parameters Set.vi"("SGamma Parameters"=w1908, "error in (no error)"=w1920, "XPS error in (no error)"=w1921, "Positioner Name (250 c max)"=w1916, "connection ID in"=w1922) -> ("error out"=w1915:errorcluster, "XPS error out"=w1914:errorcluster, "connection ID out"=w1918:T9)  [unwired: 4 in]
              }
              frame #1 {
                n771 = local read "X travel"() -> (w1929:dbl)
                n772 = local read "Y travel"() -> (w1928:dbl)
                n773 = case shown="False" w1925 {
                  tunnel: w1929 -> [w1941 w1945]
                  tunnel: w1928 -> [w1940 w1944]
                  tunnel: [w1940 w1943] -> w1927
                  tunnel: [w1941 w1942] -> w1926
                  frame False {
                  }
                  frame True {
                    n774 = Negate(x=w1945) -> (-x=w1942:dbl)
                    n775 = Negate(x=w1944) -> (-x=w1943:dbl)
                  }
                }
                n776 = call <userlib>:"Single Axis Group Move Relative.vi"("Target Displacement (units)"=w1927, "error in (no error)"=w1937, "XPS error in (no error)"=w1936, "SingleAxis Group  Name (250 c max)"=w1930, "connection ID in"=w1939) -> ("error out"=w1934:errorcluster, "XPS error out"=w1935:errorcluster, "connection ID out"=w1938:T9)  [unwired: 4 in]
                n777 = call <userlib>:"Single Axis Group Move Relative.vi"("Target Displacement (units)"=w1926, "error in (no error)"=w1934, "XPS error in (no error)"=w1935, "SingleAxis Group  Name (250 c max)"=w1931, "connection ID in"=w1938) -> ("error out"=w1932:errorcluster, "connection ID out"=w1933:T9)  [unwired: 4 in, 1 out]
                n778 = call <userlib>:"Close TCP-IP.vi"("error in (no error)"=w1932, "connection ID in"=w1933) -> ()  [unwired: 9 in, 1 out]
              }
              frame #2 {
                n779 = Wait (ms)(milliseconds to wait=u32 1000) -> ()  [unwired: 1 out]
              }
              frame #3 {
                n780 = case shown="True" w1947 {
                  tunnel: ["capture " ("string") "microscope " ("string")] -> w1948
                  frame False {
                  }
                  frame True {
                  }
                }
                n781 = Concatenate Strings("Stages translated to the " ("StringOut"), w1948, "position." ("string")) -> (w1951:string)
              }
            }
          }
        }
      }
    }
    n782 = Get Date/Time In Seconds() -> (seconds since 1Jan1904=w816:timestamp)
    n783 = Format Date/Time String(time format string (%c)="%m/%d/%y - %I:%M %p  ", seconds (now)=w816) -> (date/time string=w815:string)  [unwired: 1 in]
    n784 = Empty String/Path?(string/path=w812) -> (empty?=w814:bool)
    n785 = Concatenate Strings(w815, w812, "\r") -> (w813:string)
    n786 = case shown="False" w814 {
      tunnel: w813 -> [w822 _]
      frame False {
        n787 = invoke on="Log" class="Str" method="Append String"("string"=w822) -> (error out=w821:errorcluster)  [unwired: 3 in, 3 out]
        n788 = property on="Log" class="Str"(error in=w821, "Text.Scroll Position"=u32 500000) -> ()  [unwired: 1 in, 2 out]
      }
      frame True {
      }
    }
  }
  n789 = control-ref of="Init Camera"() -> (w74:refnum<vi>)
  n790 = control-ref of="Stop Live"() -> (w67:refnum<vi>)
  n791 = property on="Property Node" class="Bool"(reference=w67, "Disabled"=w70) -> (reference out=w58:refnum<vi>, error out=w57:errorcluster)  [unwired: 1 in]
  n792 = property on="Property Node" class="Bool"(reference=w74, "Disabled"=w73) -> (reference out=w62:refnum<vi>, error out=w61:errorcluster)  [unwired: 1 in]
  n793 = Close Reference(reference=w58, error in (no error)=w57) -> ()  [unwired: 1 out]
  n794 = Close Reference(reference=w62, error in (no error)=w61) -> ()  [unwired: 1 out]
  n795 = control-ref of="Load Parameter"() -> (w68:refnum<vi>)
  n796 = control-ref of="Start Live"() -> (w71:refnum<vi>)
  n797 = property on="Property Node" class="Bool"(reference=w71, "Disabled"=w72) -> (reference out=w60:refnum<vi>, error out=w59:errorcluster)  [unwired: 1 in]
  n798 = property on="Property Node" class="Bool"(reference=w68, "Disabled"=w69) -> (reference out=w56:refnum<vi>, error out=w55:errorcluster)  [unwired: 1 in]
  n799 = Close Reference(reference=w60, error in (no error)=w59) -> ()  [unwired: 1 out]
  n800 = Close Reference(reference=w56, error in (no error)=w55) -> ()  [unwired: 1 out]
